vi "FlexMag - 24-03-2023.vi"() -> ()   [LabVIEW 2018] (continued)
                                }
                                }
                                n17277 = local read "CH3_Trns_BP_Right_DI"() -> (w21347:bool)
                                n17278 = case shown="False" w21347 {
                                tunnel: [FALSE TRUE] -> w21346
                                frame False {
                                n17279 = Wait Until Next ms Multiple(millisecond multiple=u32 200) -> ()  [unwired: 1 out]
                                n17280 = local write "CH3_Trns_BP_Right_DO"(TRUE ("CH1_WFC_DO")) -> ()
                                }
                                frame True {
                                }
                                }
                                n17281 = local read "abort ch3"() -> (w21349:bool)
                                n17282 = local read "ch3 shutdown alg"() -> (w21351:bool)
                                n17283 = Not(x=w21351) -> (.not. x?=w21350:bool)
                                n17284 = Compound Arithmetic op=OR(w21346, w21349, w21350) -> (w21348:bool)
                                }
                              }
                            }
                          }
                        }
                      }
                      frame True {
                      }
                    }
                  }
                }
              }
              frame #20 {
                n17285 = local read "ch3 shutdown alg"() -> (w21361:bool)
                n17286 = case shown="True" w21361 {
                  frame False {
                  }
                  frame True {
                    n17287 = local read "abort ch3"() -> (w21362:bool)
                    n17288 = case shown="False" w21362 {
                      frame False {
                        n17289 = local read "ch3 vent?"() -> (w21363:bool)
                        n17290 = case shown="False" w21363 {
                          frame False {
                            n17291 = local write "ch3 sd trns bp right close led"(TRUE ("ch1 sd cc close led")) -> ()
                            n17292 = Wait (ms)(milliseconds to wait=u32 1000) -> ()  [unwired: 1 out]
                          }
                          frame True {
                            n17293 = local write "ch3 sd trns bp right open led"(TRUE ("ch1 sd cc close led")) -> ()
                            n17294 = Wait (ms)(milliseconds to wait=u32 1000) -> ()  [unwired: 1 out]
                          }
                        }
                      }
                      frame True {
                      }
                    }
                  }
                }
              }
              frame #21 {
                n17295 = local read "ch3 shutdown alg"() -> (w21368:bool)
                n17296 = case shown="True" w21368 {
                  frame False {
                  }
                  frame True {
                    n17297 = local read "abort ch3"() -> (w21369:bool)
                    n17298 = case shown="False" w21369 {
                      frame False {
                        n17299 = local read "ch3 vent?"() -> (w21370:bool)
                        n17300 = case shown="True" w21370 {
                          frame False {
                          }
                          frame True {
                            n17301 = while {
                              i -> [w21373]
                              stop <- w21376 stop-if-true
                              n17302 = Greater?(x=w21373, y=100) -> (0:w21372:bool)
                              n17303 = case shown="True" w21372 {
                                frame False {
                                }
                                frame True {
                                n17304 = local write "Warning Message"("CH3 ShutDown process  is canceled !\nCH3 CH VBV couldn't be opened" ("Warning Message")) -> ()
                                n17305 = local write "ch3 shutdown error"(TRUE ("ch1 pumpdown error")) -> ()
                                }
                              }
                              n17306 = local read "CH3_CH_VBV_DI"() -> (w21371:bool)
                              n17307 = case shown="False" w21371 {
                                tunnel: [FALSE TRUE] -> w21375
                                frame False {
                                n17308 = Wait Until Next ms Multiple(millisecond multiple=u32 200) -> ()  [unwired: 1 out]
                                n17309 = local write "CH3_CH_VBV_DO"(TRUE ("CH1_WFC_DO")) -> ()
                                }
                                frame True {
                                }
                              }
                              n17310 = local read "ch3 shutdown alg"() -> (w21377:bool)
                              n17311 = local read "abort ch3"() -> (w21379:bool)
                              n17312 = Not(x=w21377) -> (.not. x?=w21378:bool)
                              n17313 = Compound Arithmetic op=OR(w21375, w21379, w21378) -> (w21376:bool)
                            }
                          }
                        }
                      }
                      frame True {
                      }
                    }
                  }
                }
              }
              frame #22 {
                n17314 = local read "ch3 shutdown alg"() -> (w21386:bool)
                n17315 = case shown="True" w21386 {
                  frame False {
                  }
                  frame True {
                    n17316 = local read "abort ch3"() -> (w21387:bool)
                    n17317 = case shown="False" w21387 {
                      frame False {
                        n17318 = local read "ch3 vent?"() -> (w21388:bool)
                        n17319 = case shown="True" w21388 {
                          frame False {
                          }
                          frame True {
                            n17320 = local write "ch3 sd ch vbv open led"(TRUE ("ch1 sd cc close led")) -> ()
                            n17321 = Wait (ms)(milliseconds to wait=u32 1000) -> ()  [unwired: 1 out]
                          }
                        }
                      }
                      frame True {
                      }
                    }
                  }
                }
              }
              frame #23 {
                n17322 = local read "ch3 shutdown alg"() -> (w21391:bool)
                n17323 = case shown="True" w21391 {
                  frame False {
                  }
                  frame True {
                    n17324 = local read "abort ch3"() -> (w21392:bool)
                    n17325 = case shown="False" w21392 {
                      frame False {
                        n17326 = local read "ch3 vent?"() -> (w21393:bool)
                        n17327 = case shown="True" w21393 {
                          frame False {
                            n17328 = while {
                              i -> [w21400]
                              stop <- w21396 stop-if-true
                              # "10min"
                              n17329 = Greater Or Equal?(x=w21400, y=3000) -> (x >= y?=w21402:bool)
                              n17330 = case shown="True" w21402 {
                                frame False {
                                }
                                frame True {
                                n17331 = local write "ch3 shutdown error"(TRUE ("ch1 pumpdown error")) -> ()
                                n17332 = local write "Warning Message"("CH3 ShutDown process  is canceled !\nCH3 PL ATM switch  couldn't be opened" ("Warning Message")) -> ()
                                }
                              }
                              n17333 = local read "CH3_PL_ATM_DI"() -> (w21394:bool)
                              n17334 = local read "abort ch3"() -> (w21397:bool)
                              n17335 = local read "ch3 shutdown alg"() -> (w21399:bool)
                              n17336 = case shown="True" w21394 {
                                tunnel: [FALSE TRUE] -> w21395
                                frame False {
                                n17337 = Wait Until Next ms Multiple(millisecond multiple=u32 200) -> ()  [unwired: 1 out]
                                }
                                frame True {
                                }
                              }
                              n17338 = Not(x=w21399) -> (.not. x?=w21398:bool)
                              n17339 = Compound Arithmetic op=OR(w21395, w21397, w21398) -> (w21396:bool)
                            }
                          }
                          frame True {
                            n17340 = while {
                              i -> [w21416]
                              stop <- w21412 stop-if-true
                              # "10min"
                              n17341 = Greater Or Equal?(x=w21416, y=3000) -> (x >= y?=w21418:bool)
                              n17342 = case shown="True" w21418 {
                                frame False {
                                }
                                frame True {
                                n17343 = local write "ch3 shutdown error"(TRUE ("ch1 pumpdown error")) -> ()
                                n17344 = local write "Warning Message"("CH2 ShutDown process  is canceled !\nCH2 ATM switches  couldn't be opened" ("Warning Message")) -> ()
                                }
                              }
                              n17345 = local read "CH3_CH_ATM_DI"() -> (w21410:bool)
                              n17346 = local read "CH3_PL_ATM_DI"() -> (w21409:bool)
                              n17347 = And(x=w21410, y=w21409) -> (x .and. y?=w21408:bool)
                              n17348 = local read "abort ch3"() -> (w21413:bool)
                              n17349 = local read "ch3 shutdown alg"() -> (w21415:bool)
                              n17350 = case shown="False" w21408 {
                                tunnel: [FALSE TRUE] -> w21411
                                frame False {
                                n17351 = Wait Until Next ms Multiple(millisecond multiple=u32 200) -> ()  [unwired: 1 out]
                                }
                                frame True {
                                }
                              }
                              n17352 = Not(x=w21415) -> (.not. x?=w21414:bool)
                              n17353 = Compound Arithmetic op=OR(w21411, w21413, w21414) -> (w21412:bool)
                            }
                          }
                        }
                      }
                      frame True {
                      }
                    }
                  }
                }
              }
              frame #24 {
                n17354 = local read "ch3 shutdown alg"() -> (w21424:bool)
                n17355 = case shown="True" w21424 {
                  frame False {
                  }
                  frame True {
                    n17356 = local read "abort ch3"() -> (w21425:bool)
                    n17357 = case shown="False" w21425 {
                      frame False {
                        n17358 = local read "ch3 vent?"() -> (w21426:bool)
                        n17359 = case shown="True" w21426 {
                          frame False {
                            n17360 = local write "ch3 sd PL atm on led"(TRUE ("ch1 sd cc close led")) -> ()
                            n17361 = Wait (ms)(milliseconds to wait=u32 1000) -> ()  [unwired: 1 out]
                          }
                          frame True {
                            w21429 = FALSE ("pcgv3 auto close")
                            w21431 = "ATMOSPHERE" ("ch3_4 vacuum level")
                            n17362 = local write "pcgv3 auto close"(TRUE ("pcgv3 auto close")) -> ()
                            n17363 = local write "CH3_Trns_BP_Right_DO"(w21429) -> ()
                            n17364 = local write "CH3_Trns_BP_Left_DO"(w21429) -> ()
                            n17365 = local write "ch3 sd PL-CH atm on led"(TRUE ("ch1 sd cc close led")) -> ()
                            n17366 = Wait (ms)(milliseconds to wait=u32 500) -> ()  [unwired: 1 out]
                            n17367 = local write "ch2_3 vacuum level"(w21431) -> ()
                            n17368 = local write "ch3_4 vacuum level"(w21431) -> ()
                          }
                        }
                      }
                      frame True {
                      }
                    }
                  }
                }
              }
              frame #25 {
                n17369 = local read "ch3 shutdown alg"() -> (w21434:bool)
                n17370 = case shown="True" w21434 {
                  frame False {
                  }
                  frame True {
                    n17371 = local read "abort ch3"() -> (w21435:bool)
                    n17372 = case shown="False" w21435 {
                      frame False {
                        n17373 = local read "ch3 vent?"() -> (w21436:bool)
                        n17374 = case shown="True" w21436 {
                          frame False {
                            w21439 = TRUE ("Buzzer DO")
                            n17375 = local write "Buzzer DO"(w21439) -> ()
                            n17376 = local write "ch3 sd completed led"(w21439) -> ()
                            n17377 = Wait (ms)(milliseconds to wait=u32 3000) -> ()  [unwired: 1 out]
                            n17378 = local write "System Status"("CH3 SHUTDOWN PROCESS COMPLETED" ("System Status")) -> ()
                          }
                          frame True {
                            w21440 = TRUE ("Buzzer DO")
                            n17379 = local write "Buzzer DO"(w21440) -> ()
                            n17380 = local write "ch3 sd completed led"(w21440) -> ()
                            n17381 = Wait (ms)(milliseconds to wait=u32 3000) -> ()  [unwired: 1 out]
                            n17382 = local write "System Status"("CH3 VENT PROCESS COMPLETED" ("System Status")) -> ()
                          }
                        }
                      }
                      frame True {
                      }
                    }
                  }
                }
              }
              frame #26 {
                n17383 = local read "ch3 shutdown alg"() -> (w21443:bool)
                n17384 = case shown="True" w21443 {
                  frame False {
                  }
                  frame True {
                    n17385 = local read "abort ch3"() -> (w21444:bool)
                    n17386 = case shown="False" w21444 {
                      frame False {
                        w21446 = FALSE ("Buzzer DO")
                        n17387 = local write "Buzzer DO"(w21446) -> ()
                        n17388 = local write "ch3 shutdown alg"(w21446) -> ()
                        n17389 = local write "Shut Down CH3"(w21446) -> ()
                        n17390 = Wait (ms)(milliseconds to wait=u32 3000) -> ()  [unwired: 1 out]
                        n17391 = local write "System Status"("SEMI-AUTOMATIC MODE " ("System Status")) -> ()
                      }
                      frame True {
                      }
                    }
                  }
                }
              }
            }
          }
          frame True {
          }
        }
      }
    }
  }
  n17392 = while {
    stop <- FALSE stop-if-true
    n17393 = Wait Until Next ms Multiple(millisecond multiple=u32 300) -> ()  [unwired: 1 out]
    n17394 = case shown="True" "ch1 pumpdown alg" {
      frame False {
      }
      frame True {
        n17395 = local read "abort ch1"() -> (w22330:bool)
        n17396 = case shown="False" w22330 {
          frame False {
            n17397 = stacked-sequence {
              frame #0 {
                n17398 = stacked-sequence {
                  frame #0 {
                    n17399 = local write "ch1 pd clear"(TRUE ("ch1 pd clear")) -> ()
                    n17400 = Wait (ms)(milliseconds to wait=u32 100) -> ()  [unwired: 1 out]
                  }
                  frame #1 {
                    # "ar"
                  }
                  frame #2 {
                    n17401 = local write "System Status"("CH1 PUMPDOWN PROCESS IN PROGRESS" ("System Status")) -> ()
                  }
                  frame #3 {
                    n17402 = local read "CH1_DS_DI"() -> (w22334:bool)
                    n17403 = case shown="False" w22334 {
                      frame False {
                        n17404 = stacked-sequence {
                          frame #0 {
                            n17405 = local write "Buzzer DO"(TRUE ("Buzzer DO")) -> ()
                            n17406 = Wait (ms)(milliseconds to wait=u32 100) -> ()  [unwired: 1 out]
                          }
                          frame #1 {
                            n17407 = while {
                              i -> [w22339]
                              stop <- w22342 stop-if-true
                              n17408 = Greater?(x=w22339, y=900) -> (0:w22338:bool)
                              n17409 = case shown="True" w22338 {
                                frame False {
                                }
                                frame True {
                                n17410 = local write "Warning Message"("CH1 PumpDown process  is canceled !\nCH1 Door is open" ("Warning Message")) -> ()
                                n17411 = local write "ch1 pumpdown error"(TRUE ("ch1 pumpdown error")) -> ()
                                }
                              }
                              n17412 = local read "CH1_DS_DI"() -> (w22337:bool)
                              n17413 = case shown="True" w22337 {
                                tunnel: [FALSE TRUE] -> w22341
                                frame False {
                                n17414 = Wait Until Next ms Multiple(millisecond multiple=u32 200) -> ()  [unwired: 1 out]
                                }
                                frame True {
                                n17415 = local write "Buzzer DO"(FALSE ("Buzzer DO")) -> ()
                                }
                              }
                              n17416 = local read "ch1 pumpdown alg"() -> (w22343:bool)
                              n17417 = local read "abort ch1"() -> (w22345:bool)
                              n17418 = Not(x=w22343) -> (.not. x?=w22344:bool)
                              n17419 = Compound Arithmetic op=OR(w22341, w22345, w22344) -> (w22342:bool)
                            }
                          }
                        }
                      }
                      frame True {
                      }
                    }
                  }
                  frame #4 {
                    n17420 = disable-structure shown="Disabled" {
                      frame Disabled {
                        n17421 = while {
                          i -> [w22354]
                          stop <- w22357 stop-if-true
                          n17422 = Greater?(x=w22354, y=900) -> (0:w22353:bool)
                          n17423 = case shown="True" w22353 {
                            frame False {
                            }
                            frame True {
                              n17424 = local write "Warning Message"("CH1 PumpDown process  is canceled !\nCH1 Water Switch couldn't be opened" ("Warning Message")) -> ()
                              n17425 = local write "ch1 pumpdown error"(TRUE ("ch1 pumpdown error")) -> ()
                            }
                          }
                          n17426 = local read "CH1_WFC_DI"() -> (w22352:bool)
                          n17427 = case shown="True" w22352 {
                            tunnel: [FALSE TRUE] -> w22356
                            frame False {
                              n17428 = Wait Until Next ms Multiple(millisecond multiple=u32 200) -> ()  [unwired: 1 out]
                              n17429 = local write "CH1_WFC_DO"(TRUE ("CH1_WFC_DO")) -> ()
                            }
                            frame True {
                            }
                          }
                          n17430 = local read "ch1 pumpdown alg"() -> (w22358:bool)
                          n17431 = local read "abort ch1"() -> (w22360:bool)
                          n17432 = Not(x=w22358) -> (.not. x?=w22359:bool)
                          n17433 = Compound Arithmetic op=OR(w22356, w22360, w22359) -> (w22357:bool)
                        }
                      }
                      frame Enabled {
                      }
                    }
                  }
                }
              }
              frame #1 {
                # "ATM switches close"
                n17434 = local read "ch1 pumpdown alg"() -> (w22367:bool)
                n17435 = case shown="True" w22367 {
                  frame False {
                  }
                  frame True {
                    n17436 = local read "abort ch1"() -> (w22368:bool)
                    n17437 = case shown="False" w22368 {
                      frame False {
                        w22370 = FALSE ("CH1_PL_ATM_DO")
                        n17438 = local write "CH1_PL_ATM_DO"(w22370) -> ()
                        n17439 = local write "CH1_CH_ATM_DO"(w22370) -> ()
                        n17440 = Wait (ms)(milliseconds to wait=u32 3000) -> ()  [unwired: 1 out]
                      }
                      frame True {
                      }
                    }
                  }
                }
              }
              frame #2 {
                n17441 = local read "ch1 pumpdown alg"() -> (w22371:bool)
                n17442 = case shown="True" w22371 {
                  frame False {
                  }
                  frame True {
                    n17443 = local read "abort ch1"() -> (w22372:bool)
                    n17444 = case shown="False" w22372 {
                      frame False {
                        n17445 = local write "ch1 atms close led"(TRUE ("CH1_PL_ATM_DO")) -> ()
                        n17446 = Wait (ms)(milliseconds to wait=u32 1000) -> ()  [unwired: 1 out]
                      }
                      frame True {
                      }
                    }
                  }
                }
              }
              frame #3 {
                # "ch vbv close"
                n17447 = local read "ch1 pumpdown alg"() -> (w22375:bool)
                n17448 = case shown="True" w22375 {
                  frame False {
                  }
                  frame True {
                    n17449 = local read "abort ch1"() -> (w22376:bool)
                    n17450 = case shown="False" w22376 {
                      frame False {
                        n17451 = while {
                          i -> [w22379]
                          stop <- w22382 stop-if-true
                          n17452 = Greater Or Equal?(x=w22379, y=100) -> (x >= y?=w22380:bool)
                          n17453 = case shown="True" w22380 {
                            frame False {
                            }
                            frame True {
                              n17454 = local write "Warning Message"("CH1 PumpDown process  is canceled !\nCH1 CH VBV couldn't be closed" ("Warning Message")) -> ()
                              n17455 = local write "ch1 pumpdown error"(TRUE ("ch1 pumpdown error")) -> ()
                            }
                          }
                          n17456 = local read "CH1_CH_VBV_DI"() -> (w22377:bool)
                          n17457 = local read "ch1 pumpdown alg"() -> (w22385:bool)
                          n17458 = case shown="True" w22377 {
                            tunnel: [TRUE FALSE] -> w22381
                            frame False {
                            }
                            frame True {
                              n17459 = local write "CH1_CH_VBV_DO"(FALSE ("CH1_CH_VBV_DO")) -> ()
                              n17460 = Wait Until Next ms Multiple(millisecond multiple=u32 200) -> ()  [unwired: 1 out]
                            }
                          }
                          n17461 = local read "abort ch1"() -> (w22383:bool)
                          n17462 = Not(x=w22385) -> (.not. x?=w22384:bool)
                          n17463 = Compound Arithmetic op=OR(w22381, w22383, w22384) -> (w22382:bool)
                        }
                      }
                      frame True {
                      }
                    }
                  }
                }
              }
              frame #4 {
                n17464 = local read "ch1 pumpdown alg"() -> (w22392:bool)
                n17465 = case shown="True" w22392 {
                  frame False {
                  }
                  frame True {
                    n17466 = local read "abort ch1"() -> (w22393:bool)
                    n17467 = case shown="False" w22393 {
                      frame False {
                        n17468 = local write "ch1 ch vbv close led"(TRUE ("ch1 ch vbv close")) -> ()
                        n17469 = Wait (ms)(milliseconds to wait=u32 1000) -> ()  [unwired: 1 out]
                      }
                      frame True {
                      }
                    }
                  }
                }
              }
              frame #5 {
                # "pl vbv close"
                n17470 = local read "ch1 pumpdown alg"() -> (w22396:bool)
                n17471 = case shown="True" w22396 {
                  frame False {
                  }
                  frame True {
                    n17472 = local read "abort ch1"() -> (w22397:bool)
                    n17473 = case shown="False" w22397 {
                      frame False {
                        n17474 = while {
                          i -> [w22400]
                          stop <- w22403 stop-if-true
                          n17475 = Greater Or Equal?(x=w22400, y=100) -> (x >= y?=w22401:bool)
                          n17476 = case shown="True" w22401 {
                            frame False {
                            }
                            frame True {
                              n17477 = local write "Warning Message"("CH1 PumpDown process  is canceled !\nCH1 PL VBV couldn't be closed" ("Warning Message")) -> ()
                              n17478 = local write "ch1 pumpdown error"(TRUE ("ch1 pumpdown error")) -> ()
                            }
                          }
                          n17479 = local read "CH1_PL_VBV_DI"() -> (w22398:bool)
                          n17480 = local read "ch1 pumpdown alg"() -> (w22406:bool)
                          n17481 = case shown="True" w22398 {
                            tunnel: [TRUE FALSE] -> w22402
                            frame False {
                            }
                            frame True {
                              n17482 = Wait Until Next ms Multiple(millisecond multiple=u32 200) -> ()  [unwired: 1 out]
                              n17483 = local write "CH1_PL_VBV_DO"(FALSE ("CH1_CH_VBV_DO")) -> ()
                            }
                          }
                          n17484 = local read "abort ch1"() -> (w22404:bool)
                          n17485 = Not(x=w22406) -> (.not. x?=w22405:bool)
                          n17486 = Compound Arithmetic op=OR(w22402, w22404, w22405) -> (w22403:bool)
                        }
                      }
                      frame True {
                      }
                    }
                  }
                }
              }
              frame #6 {
                n17487 = local read "ch1 pumpdown alg"() -> (w22413:bool)
                n17488 = case shown="True" w22413 {
                  frame False {
                  }
                  frame True {
                    n17489 = local read "abort ch1"() -> (w22414:bool)
                    n17490 = case shown="False" w22414 {
                      frame False {
                        n17491 = local write "ch1 pl vbv close led"(TRUE ("ch1 ch vbv close")) -> ()
                        n17492 = Wait (ms)(milliseconds to wait=u32 1000) -> ()  [unwired: 1 out]
                      }
                      frame True {
                      }
                    }
                  }
                }
              }
              frame #7 {
                n17493 = local read "ch1 pumpdown alg"() -> (w22417:bool)
                n17494 = case shown="True" w22417 {
                  frame False {
                  }
                  frame True {
                    n17495 = local read "abort ch1"() -> (w22418:bool)
                    n17496 = case shown="False" w22418 {
                      frame False {
                        n17497 = local read "ch2 ch pg torr"() -> (w22422:dbl)
                        n17498 = local read "CH1_CH_ATM_DI"() -> (w22420:bool)
                        n17499 = Less?(x=w22422, y=0.5) -> (x < y?=w22421:bool)
                        n17500 = And(x=w22420, y=w22421) -> (x .and. y?=w22419:bool)
                        n17501 = case shown="True" w22419 {
                          frame False {
                            # "ch trns bp left close"
                            n17502 = while {
                              i -> [w22426]
                              stop <- w22429 stop-if-true
                              n17503 = Greater Or Equal?(x=w22426, y=100) -> (x >= y?=w22427:bool)
                              n17504 = case shown="True" w22427 {
                                frame False {
                                }
                                frame True {
                                n17505 = local write "Warning Message"("CH1 PumpDown process  is canceled !\nCH1 TRNS BP Left couldn't be closed" ("Warning Message")) -> ()
                                n17506 = local write "ch1 pumpdown error"(TRUE ("ch1 pumpdown error")) -> ()
                                }
                              }
                              n17507 = local read "CH1_Trns_BP_Left_DI"() -> (w22424:bool)
                              n17508 = local read "ch1 pumpdown alg"() -> (w22432:bool)
                              n17509 = case shown="True" w22424 {
                                tunnel: [TRUE FALSE] -> w22428
                                frame False {
                                }
                                frame True {
                                n17510 = local write "CH1_Trns_BP_Left_DO"(FALSE ("CH1_CH_VBV_DO")) -> ()
                                n17511 = Wait Until Next ms Multiple(millisecond multiple=u32 200) -> ()  [unwired: 1 out]
                                }
                              }
                              n17512 = local read "abort ch1"() -> (w22430:bool)
                              n17513 = Not(x=w22432) -> (.not. x?=w22431:bool)
                              n17514 = Compound Arithmetic op=OR(w22428, w22430, w22431) -> (w22429:bool)
                            }
                          }
                          frame True {
                            # "ch trns bp left open"
                            n17515 = while {
                              i -> [w22441]
                              stop <- w22444 stop-if-true
                              n17516 = Greater Or Equal?(x=w22441, y=100) -> (x >= y?=w22442:bool)
                              n17517 = case shown="True" w22442 {
                                frame False {
                                }
                                frame True {
                                n17518 = local write "Warning Message"("CH1 PumpDown process  is canceled !\nCH1 TRNS BP Left couldn't be opened" ("Warning Message")) -> ()
                                n17519 = local write "ch1 pumpdown error"(TRUE ("ch1 pumpdown error")) -> ()
                                }
                              }
                              n17520 = local read "CH1_Trns_BP_Left_DI"() -> (w22439:bool)
                              n17521 = local read "ch1 pumpdown alg"() -> (w22447:bool)
                              n17522 = case shown="False" w22439 {
                                tunnel: [FALSE TRUE] -> w22443
                                frame False {
                                n17523 = local write "CH1_Trns_BP_Left_DO"(TRUE ("CH1_CH_VBV_DO")) -> ()
                                n17524 = Wait Until Next ms Multiple(millisecond multiple=u32 200) -> ()  [unwired: 1 out]
                                }
                                frame True {
                                }
                              }
                              n17525 = local read "abort ch1"() -> (w22445:bool)
                              n17526 = Not(x=w22447) -> (.not. x?=w22446:bool)
                              n17527 = Compound Arithmetic op=OR(w22443, w22445, w22446) -> (w22444:bool)
                            }
                          }
                        }
                      }
                      frame True {
                      }
                    }
                  }
                }
              }
              frame #8 {
                n17528 = local read "ch1 pumpdown alg"() -> (w22454:bool)
                n17529 = case shown="True" w22454 {
                  frame False {
                  }
                  frame True {
                    n17530 = local read "abort ch1"() -> (w22455:bool)
                    n17531 = case shown="False" w22455 {
                      frame False {
                        n17532 = local read "CH1_Trns_BP_Left_DI"() -> (w22456:bool)
                        n17533 = case shown="True" w22456 {
                          frame False {
                          }
                          frame True {
                            n17534 = local write "ch1 trns bp left close led"(TRUE ("ch1 ch vbv close")) -> ()
                            n17535 = Wait (ms)(milliseconds to wait=u32 1000) -> ()  [unwired: 1 out]
                          }
                        }
                      }
                      frame True {
                      }
                    }
                  }
                }
              }
              frame #9 {
                # "ch trns gv 1-2 close"
                n17536 = local read "ch1 pumpdown alg"() -> (w22459:bool)
                n17537 = case shown="True" w22459 {
                  frame False {
                  }
                  frame True {
                    n17538 = local read "abort ch1"() -> (w22460:bool)
                    n17539 = case shown="False" w22460 {
                      frame False {
                        n17540 = while {
                          i -> [w22463]
                          stop <- w22466 stop-if-true
                          n17541 = Greater Or Equal?(x=w22463, y=600) -> (x >= y?=w22464:bool)
                          n17542 = case shown="True" w22464 {
                            frame False {
                            }
                            frame True {
                              n17543 = local write "Warning Message"("CH1 PumpDown process  is canceled !\nCH1-CH2 TRNS GV couldn't be closed" ("Warning Message")) -> ()
                              n17544 = local write "ch1 pumpdown error"(TRUE ("ch1 pumpdown error")) -> ()
                            }
                          }
                          n17545 = local read "CH1_Trns_Gv_Close_DI"() -> (w22461:bool)
                          n17546 = case shown="False" w22461 {
                            tunnel: [FALSE TRUE] -> w22465
                            frame False {
                              n17547 = local write "CH1_Trns_Gv_Open_DO"(FALSE) -> ()
                              n17548 = local write "CH1_Trns_Gv_Close_DO"(TRUE ("CH1_CH_VBV_DO")) -> ()
                              n17549 = Wait Until Next ms Multiple(millisecond multiple=u32 200) -> ()  [unwired: 1 out]
                            }
                            frame True {
                            }
                          }
                          n17550 = local read "ch1 pumpdown alg"() -> (w22469:bool)
                          n17551 = local read "abort ch1"() -> (w22467:bool)
                          n17552 = Not(x=w22469) -> (.not. x?=w22468:bool)
                          n17553 = Compound Arithmetic op=OR(w22465, w22467, w22468) -> (w22466:bool)
                        }
                      }
                      frame True {
                      }
                    }
                  }
                }
              }
              frame #10 {
                n17554 = local read "ch1 pumpdown alg"() -> (w22477:bool)
                n17555 = case shown="True" w22477 {
                  frame False {
                  }
                  frame True {
                    n17556 = local read "abort ch1"() -> (w22478:bool)
                    n17557 = case shown="False" w22478 {
                      frame False {
                        n17558 = local write "ch1-ch2 trns gv close led 2"(TRUE ("ch1 ch vbv close")) -> ()
                        n17559 = Wait (ms)(milliseconds to wait=u32 1000) -> ()  [unwired: 1 out]
                      }
                      frame True {
                      }
                    }
                  }
                }
              }
              frame #11 {
                # "tp bv open\npc gv open"
                n17560 = local read "ch1 pumpdown alg"() -> (w22481:bool)
                n17561 = case shown="True" w22481 {
                  frame False {
                  }
                  frame True {
                    n17562 = local read "abort ch1"() -> (w22482:bool)
                    n17563 = case shown="False" w22482 {
                      frame False {
                        n17564 = local read "CH1_CH_ATM_DI"() -> (w22484:bool)
                        n17565 = local read "CH1_PL_ATM_DI"() -> (w22485:bool)
                        n17566 = And(x=w22484, y=w22485) -> (x .and. y?=w22483:bool)
                        n17567 = case shown="True" w22483 {
                          frame False {
                          }
                          frame True {
                            n17568 = stacked-sequence {
                              frame #0 {
                                # "tp bv open\npc gv open"
                              }
                              frame #1 {
                                n17569 = while {
                                i -> [w22488]
                                stop <- w22491 stop-if-true
                                n17570 = Greater Or Equal?(x=w22488, y=100) -> (x >= y?=w22489:bool)
                                n17571 = case shown="True" w22489 {
                                frame False {
                                }
                                frame True {
                                n17572 = local write "Warning Message"("CH1 PumpDown process  is canceled !\nCH1 TP BV couldn't be opened" ("Warning Message")) -> ()
                                n17573 = local write "ch1 pumpdown error"(TRUE ("ch1 pumpdown error")) -> ()
                                }
                                }
                                n17574 = local read "CH1_TP_BV_DI"() -> (w22486:bool)
                                n17575 = local read "ch1 pumpdown alg"() -> (w22494:bool)
                                n17576 = case shown="False" w22486 {
                                tunnel: [FALSE TRUE] -> w22490
                                frame False {
                                n17577 = Wait Until Next ms Multiple(millisecond multiple=u32 200) -> ()  [unwired: 1 out]
                                n17578 = local write "CH1_TP_BV_DO"(TRUE ("CH1_CH_VBV_DO")) -> ()
                                }
                                frame True {
                                }
                                }
                                n17579 = local read "abort ch1"() -> (w22492:bool)
                                n17580 = Not(x=w22494) -> (.not. x?=w22493:bool)
                                n17581 = Compound Arithmetic op=OR(w22490, w22492, w22493) -> (w22491:bool)
                                }
                              }
                              frame #2 {
                                n17582 = local read "ch1 pumpdown alg"() -> (w22501:bool)
                                n17583 = case shown="True" w22501 {
                                frame False {
                                }
                                frame True {
                                n17584 = local write "ch1 tp bv open led"(TRUE ("ch1 tp bv open led")) -> ()
                                n17585 = Wait (ms)(milliseconds to wait=u32 1000) -> ()  [unwired: 1 out]
                                }
                                }
                              }
                              frame #3 {
                                n17586 = stacked-sequence {
                                frame #0 {
                                n17587 = local read "ch1 pumpdown alg"() -> (w22504:bool)
                                n17588 = case shown="True" w22504 {
                                frame False {
                                }
                                frame True {
                                n17589 = flat-sequence {
                                frame #0 {
                                n17590 = local write "pcgv1 auto open"(TRUE ("pcgv1 auto open")) -> ()
                                }
                                frame #1 {
                                n17591 = Wait (ms)(milliseconds to wait=u32 2000) -> ()  [unwired: 1 out]
                                }
                                frame #2 {
                                n17592 = local write "pcgv1 auto open"(TRUE ("pcgv1 auto open")) -> ()
                                }
                                }
                                }
                                }
                                }
                                frame #1 {
                                n17593 = while {
                                i -> [w22514]
                                stop <- w22510 stop-if-true
                                n17594 = Greater Or Equal?(x=w22514, y=200) -> (x >= y?=w22516:bool)
                                n17595 = case shown="True" w22516 {
                                frame False {
                                }
                                frame True {
                                n17596 = local write "ch1 pumpdown error"(TRUE ("ch1 pumpdown error")) -> ()
                                n17597 = local write "Warning Message"("CH1 PumpDown process  is canceled !\nCH1 PC GV couldn't be opened" ("Warning Message")) -> ()
                                }
                                }
                                n17598 = local read "ch1 pumpdown alg"() -> (w22513:bool)
                                n17599 = local read "ch1_pcgv_gui"() -> (w22509:bool)
                                n17600 = local read "abort ch1"() -> (w22511:bool)
                                n17601 = Wait Until Next ms Multiple(millisecond multiple=u32 200) -> ()  [unwired: 1 out]
                                n17602 = Not(x=w22513) -> (.not. x?=w22512:bool)
                                n17603 = Compound Arithmetic op=OR(w22509, w22511, w22512) -> (w22510:bool)
                                }
                                }
                                }
                              }
                              frame #4 {
                                n17604 = local read "ch1 pumpdown alg"() -> (w22519:bool)
                                n17605 = case shown="True" w22519 {
                                frame False {
                                }
                                frame True {
                                n17606 = local write "ch1 pc gv open led"(TRUE ("ch1 tp bv open led")) -> ()
                                n17607 = Wait (ms)(milliseconds to wait=u32 1000) -> ()  [unwired: 1 out]
                                }
                                }
                              }
                            }
                          }
                        }
                      }
                      frame True {
                      }
                    }
                  }
                }
              }
              frame #12 {
                n17608 = stacked-sequence {
                  frame #0 {
                    n17609 = local read "ch1 pumpdown alg"() -> (w22522:bool)
                    n17610 = case shown="True" w22522 {
                      frame False {
                      }
                      frame True {
                        n17611 = local read "abort ch1"() -> (w22523:bool)
                        n17612 = case shown="False" w22523 {
                          frame False {
                            n17613 = local write "CH1_PL_ATM_DO"(TRUE ("CH1_PL_ATM_DO")) -> ()
                            n17614 = Wait (ms)(milliseconds to wait=u32 2000) -> ()  [unwired: 1 out]
                          }
                          frame True {
                          }
                        }
                      }
                    }
                  }
                  frame #1 {
                    n17615 = local read "ch1 pumpdown alg"() -> (w22526:bool)
                    n17616 = case shown="True" w22526 {
                      frame False {
                      }
                      frame True {
                        n17617 = local read "abort ch1"() -> (w22527:bool)
                        n17618 = case shown="False" w22527 {
                          frame False {
                            n17619 = local write "CH1_CH_ATM_DO"(TRUE ("CH1_CH_ATM_DO")) -> ()
                            n17620 = Wait (ms)(milliseconds to wait=u32 2000) -> ()  [unwired: 1 out]
                          }
                          frame True {
                          }
                        }
                      }
                    }
                  }
                }
              }
              frame #13 {
                # "mp start"
                n17621 = local read "ch1 pumpdown alg"() -> (w22530:bool)
                n17622 = case shown="True" w22530 {
                  frame False {
                  }
                  frame True {
                    n17623 = local read "abort ch1"() -> (w22531:bool)
                    n17624 = case shown="False" w22531 {
                      frame False {
                        n17625 = while {
                          i -> [w22536]
                          stop <- w22540 stop-if-true
                          n17626 = Greater?(x=w22536, y=100) -> (0:w22532:bool)
                          n17627 = case shown="True" w22532 {
                            frame False {
                            }
                            frame True {
                              n17628 = local write "Warning Message"("CH1 PumpDown process  is canceled !\nCH1 MP couldn't be started" ("Warning Message")) -> ()
                              n17629 = local write "ch1 pumpdown error"(TRUE ("ch1 pumpdown error")) -> ()
                            }
                          }
                          n17630 = local read "CH1_MP_DI"() -> (w22534:bool)
                          n17631 = case shown="False" w22534 {
                            tunnel: [FALSE TRUE] -> w22533
                            frame False {
                              n17632 = Wait Until Next ms Multiple(millisecond multiple=u32 200) -> ()  [unwired: 1 out]
                              n17633 = local write "CH1_MP_DO"(TRUE ("CH1_MP_DO")) -> ()
                            }
                            frame True {
                            }
                          }
                          n17634 = local read "ch1 pumpdown alg"() -> (w22539:bool)
                          n17635 = local read "abort ch1"() -> (w22537:bool)
                          n17636 = Not(x=w22539) -> (.not. x?=w22538:bool)
                          n17637 = Compound Arithmetic op=OR(w22533, w22537, w22538) -> (w22540:bool)
                        }
                      }
                      frame True {
                      }
                    }
                  }
                }
              }
              frame #14 {
                n17638 = local read "ch1 pumpdown alg"() -> (w22547:bool)
                n17639 = case shown="True" w22547 {
                  frame False {
                  }
                  frame True {
                    n17640 = local read "abort ch1"() -> (w22548:bool)
                    n17641 = case shown="False" w22548 {
                      frame False {
                        n17642 = local write "ch1 mp start led"(TRUE ("ch1 ch vbv close")) -> ()
                        n17643 = Wait (ms)(milliseconds to wait=u32 1000) -> ()  [unwired: 1 out]
                      }
                      frame True {
                      }
                    }
                  }
                }
              }
              frame #15 {
                # "pl pg check"
                n17644 = local read "ch1 pumpdown alg"() -> (w22551:bool)
                n17645 = case shown="True" w22551 {
                  frame False {
                  }
                  frame True {
                    n17646 = local read "abort ch1"() -> (w22552:bool)
                    n17647 = case shown="False" w22552 {
                      frame False {
                        n17648 = while {
                          i -> [w22559]
                          stop <- w22563 stop-if-true
                          # "30 min"
                          n17649 = Greater?(x=w22559, y=9000) -> (0:w22556:bool)
                          n17650 = case shown="True" w22556 {
                            frame False {
                            }
                            frame True {
                              n17651 = local write "Warning Message"("CH1 PumpDown process  is canceled !\nCH1 PL Pressure couldn't be reached under 0.5 Torr" ("Warning Message")) -> ()
                              n17652 = local write "ch1 pumpdown error"(TRUE ("ch1 pumpdown error")) -> ()
                            }
                          }
                          n17653 = local read "ch1 pl pg  torr"() -> (w22555:dbl)
                          n17654 = Less?(x=w22555, y=0.7) -> (x < y?=w22553:bool)
                          n17655 = case shown="False" w22553 {
                            tunnel: [FALSE TRUE] -> w22557
                            frame False {
                              n17656 = Wait Until Next ms Multiple(millisecond multiple=u32 200) -> ()  [unwired: 1 out]
                            }
                            frame True {
                            }
                          }
                          n17657 = local read "ch1 pumpdown alg"() -> (w22562:bool)
                          n17658 = local read "abort ch1"() -> (w22560:bool)
                          n17659 = Not(x=w22562) -> (.not. x?=w22561:bool)
                          n17660 = Compound Arithmetic op=OR(w22557, w22560, w22561) -> (w22563:bool)
                        }
                      }
                      frame True {
                      }
                    }
                  }
                }
              }
              frame #16 {
                n17661 = local read "ch1 pumpdown alg"() -> (w22569:bool)
                n17662 = case shown="True" w22569 {
                  frame False {
                  }
                  frame True {
                    n17663 = local read "abort ch1"() -> (w22570:bool)
                    n17664 = case shown="False" w22570 {
                      frame False {
                        n17665 = local write "ch1 pl press under 0.05 T led"(TRUE ("ch1 ch vbv close")) -> ()
                        n17666 = Wait (ms)(milliseconds to wait=u32 1000) -> ()  [unwired: 1 out]
                      }
                      frame True {
                      }
                    }
                  }
                }
              }
              frame #17 {
                # "tp bv open"
                n17667 = local read "ch1 pumpdown alg"() -> (w22573:bool)
                n17668 = case shown="True" w22573 {
                  frame False {
                  }
                  frame True {
                    n17669 = local read "abort ch1"() -> (w22574:bool)
                    n17670 = case shown="False" w22574 {
                      frame False {
                        n17671 = while {
                          i -> [w22579]
                          stop <- w22583 stop-if-true
                          n17672 = Greater?(x=w22579, y=100) -> (0:w22575:bool)
                          n17673 = case shown="True" w22575 {
                            frame False {
                            }
                            frame True {
                              n17674 = local write "Warning Message"("CH1 PumpDown process  is canceled !\nCH1 TP BV couldn't be opened" ("Warning Message")) -> ()
                              n17675 = local write "ch1 pumpdown error"(TRUE ("ch1 pumpdown error")) -> ()
                            }
                          }
                          n17676 = local read "CH1_TP_BV_DI"() -> (w22577:bool)
                          n17677 = case shown="False" w22577 {
                            tunnel: [FALSE TRUE] -> w22576
                            frame False {
                              n17678 = Wait Until Next ms Multiple(millisecond multiple=u32 200) -> ()  [unwired: 1 out]
                              n17679 = local write "CH1_TP_BV_DO"(TRUE ("CH1_MP_DO")) -> ()
                            }
                            frame True {
                            }
                          }
                          n17680 = local read "ch1 pumpdown alg"() -> (w22582:bool)
                          n17681 = local read "abort ch1"() -> (w22580:bool)
                          n17682 = Not(x=w22582) -> (.not. x?=w22581:bool)
                          n17683 = Compound Arithmetic op=OR(w22576, w22580, w22581) -> (w22583:bool)
                        }
                      }
                      frame True {
                      }
                    }
                  }
                }
              }
              frame #18 {
                n17684 = local read "ch1 pumpdown alg"() -> (w22590:bool)
                n17685 = case shown="True" w22590 {
                  frame False {
                  }
                  frame True {
                    n17686 = local read "abort ch1"() -> (w22591:bool)
                    n17687 = case shown="False" w22591 {
                      frame False {
                        n17688 = local write "ch1 tp bv open led"(TRUE ("ch1 ch vbv close")) -> ()
                        n17689 = Wait (ms)(milliseconds to wait=u32 1000) -> ()  [unwired: 1 out]
                      }
                      frame True {
                      }
                    }
                  }
                }
              }
              frame #19 {
                # "pc gv open"
                n17690 = local read "ch1 pumpdown alg"() -> (w22594:bool)
                n17691 = case shown="True" w22594 {
                  frame False {
                  }
                  frame True {
                    n17692 = local read "abort ch1"() -> (w22595:bool)
                    n17693 = case shown="False" w22595 {
                      frame False {
                        n17694 = stacked-sequence {
                          frame #0 {
                            n17695 = local read "ch1 pumpdown alg"() -> (w22596:bool)
                            n17696 = case shown="True" w22596 {
                              frame False {
                              }
                              frame True {
                                n17697 = flat-sequence {
                                frame #0 {
                                n17698 = local write "pcgv1 auto open"(TRUE ("pcgv1 auto open")) -> ()
                                }
                                frame #1 {
                                n17699 = Wait (ms)(milliseconds to wait=u32 2000) -> ()  [unwired: 1 out]
                                }
                                frame #2 {
                                n17700 = local write "pcgv1 auto open"(TRUE ("pcgv1 auto open")) -> ()
                                }
                                }
                              }